vi "RetriggerableHost_20230407.vi"() -> ()   [LabVIEW 2021]
doc: "Use this VI as a template to design an application that acquires data using advanced triggering logic from the NI PXIe-5170R/5171R."
uses:
  <instrlib>/_niInstr/Multirecord Acquisition/Interface/v1/Host/Public/Requested Record Info.ctl
  Controls/Queue_Data_Type.ctl
  <instrlib>/HSAI-RIO/Types/v1/Host/Typedefs/Temp Source.ctl
  <vilib>/FPGAPlugInAG/PXIe-5172 (8CH - 325T)/niLvFpga_Open_PXIe-5172 (8CH - 325T).vi
  <vilib>/rvi/interface/common/dynamic/niFpgaDynamicAddResources.vi
  <vilib>/FPGAPlugInAG/Dynamic/niLvFpga_Close_Dynamic.vi
  <vilib>/rvi/interface/nirviOpenFPGA/nirviOpenFPGA.xnode
  FPGA Bitfiles/Multirecord Acquisition_20220927.lvbitx
  <vilib>/rvi/interface/nirviCloseFPGA/nirviCloseFPGA.xnode
  Device Session/Device Session.lvclass
  <instrlib>/HSAI-RIO/Types/v1/Host/niHSAI Types v1 Host.lvlib
  <vilib>/Utility/TDMS File Viewer/NI_TDMS File Viewer.lvlib
  <instrlib>/_niInstr/Multirecord Acquisition/Interface/v1/Host/niInstr Multirecord Acquisition v1 Host.lvclass
panel:
  out "requested records info":T1[](array[typedef])
  in  "starting record":u64
  out "error out 2":errorcluster
  out "appended path":path
  out "Trigger":bool
  in  "trigger level lo (V)":dbl=-0.25
  in  "trigger level hi (V)":dbl=0.25
  out "actual sample rate":dbl=200000000.0 format="%#_6p"
  in  "onboard sample clock rate":dbl(ring)=200000000.0 items=["250 MHz"=250000000.0, "200 MHz"=200000000.0, "150 MHz"=150000000.0]
  in  "impedance":enum8{"Default", "1 mega ohm", "50 ohm"}(ring)=enum."50 ohm"
  in  "vertical offset (V)":dbl format="%.2p"
  out "Graph":T2(graph)
  out "fpga temperature (°C)":dbl(slide)=84.16040039062506 scale=0.0..96.0 scale format="%#_6p"
  out "power consumption (W)":dbl(slide)=28.75 scale=0.0..38.25 scale format="%#_6p"
  in  "decimation factor":u16=1
  in  "coupling":enum8{"Default", "DC", "AC"}(ring)
  in  "bandwidth":T3(ring)
  in  "pretrigger samples":u64=500
  in  "number of samples":u64=1000
  in  "RIO Device":tag="PXI1Slot2"
  in  "channel(s)":string="0,1"
  in  "vertical range (Vpp)":dbl=1.0 format="%.2p"
  out "error out":errorcluster
  in  "stop":bool
  # "RIO Device"
  # "Vertical Settings"
  # "Trigger Settings"
  # "System Monitor"
  # "Acquisition Settings"
  # "Clocking"
  # "DSP"
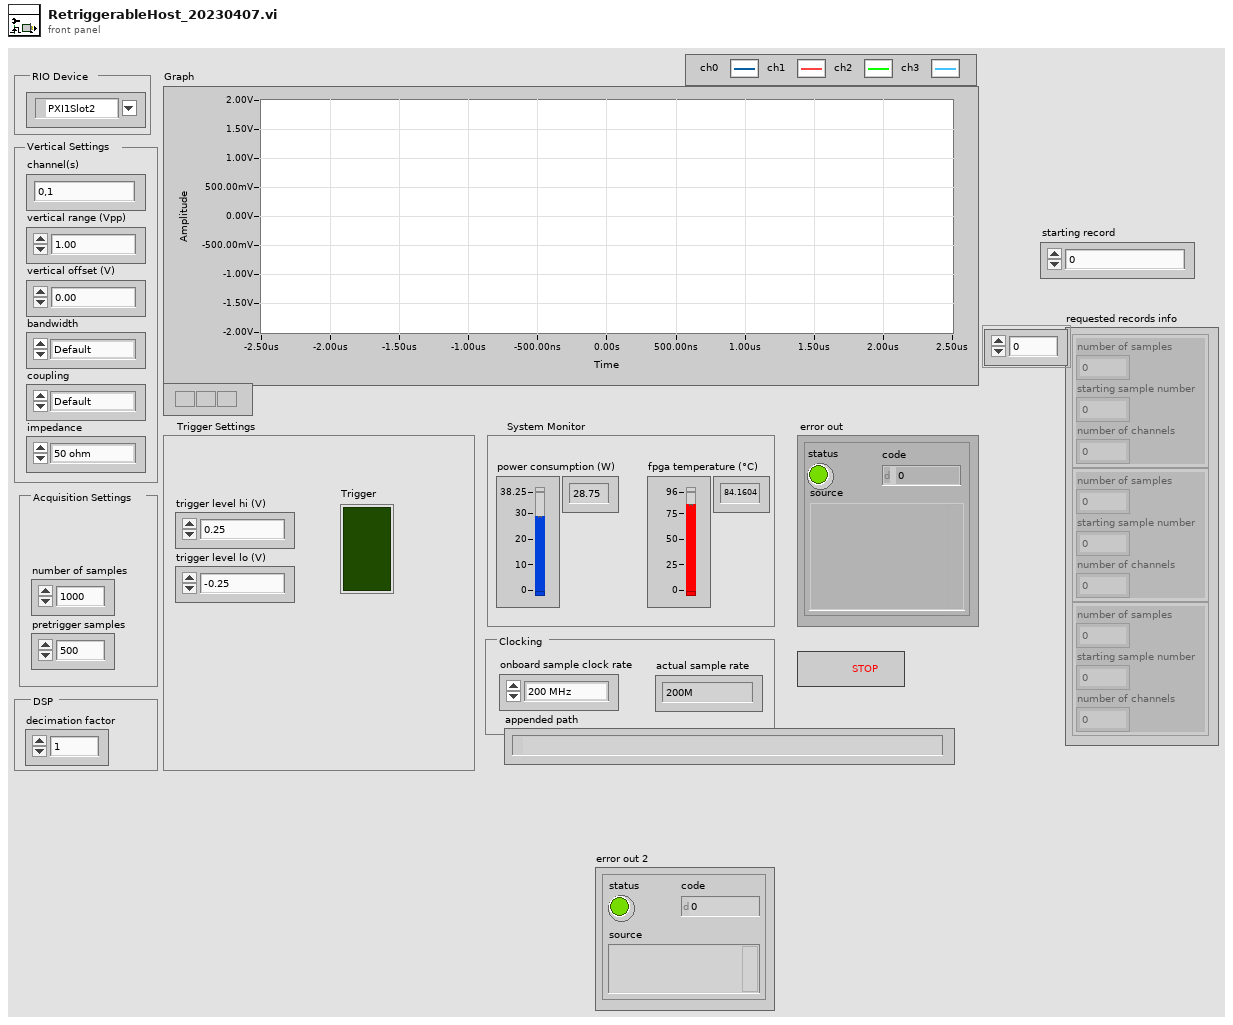
[diagram p1: front panel]
types:
  T1 = typedef "niInstr Multirecord Acquisition v1 Host.lvclass/Requested Record Info.ctl" = cluster{"number of samples":u64, "starting sample number":u64, "number of channels":u64, "timestamps":u64[]}
  T2 = cluster{"relativeX":dbl, "sample rate":dbl, "data in":dbl[]}[]
  T3 = enum8{"Default", "Full Bandwidth", "Anti-alias Filter", "80 MHz FIR Filter", "40 MHz FIR Filter", "20 MHz FIR Filter"}
  T4 = typedef "Queue_Data_Type.ctl" = cluster{"date/time string":string, "data":dbl[][]}
  T5 = enum16{"open", "open or create", "create or replace", "create", "open (read-only)"}
  T6 = enum16{"Immediate", "A", "B", "OR", "AND", "A THEN B", "B THEN A", "High Resolution"}
  T7 = typedef "niHSAI Types v1 Host.lvlib/Temp Source.ctl" = enum8{"Device Temperature", "Thermal Shutdown Margin", "FPGA Temperature", "FPGA Temperature Limit"}
  T8 = cluster{"date/time string":string, "data":dbl[][]}
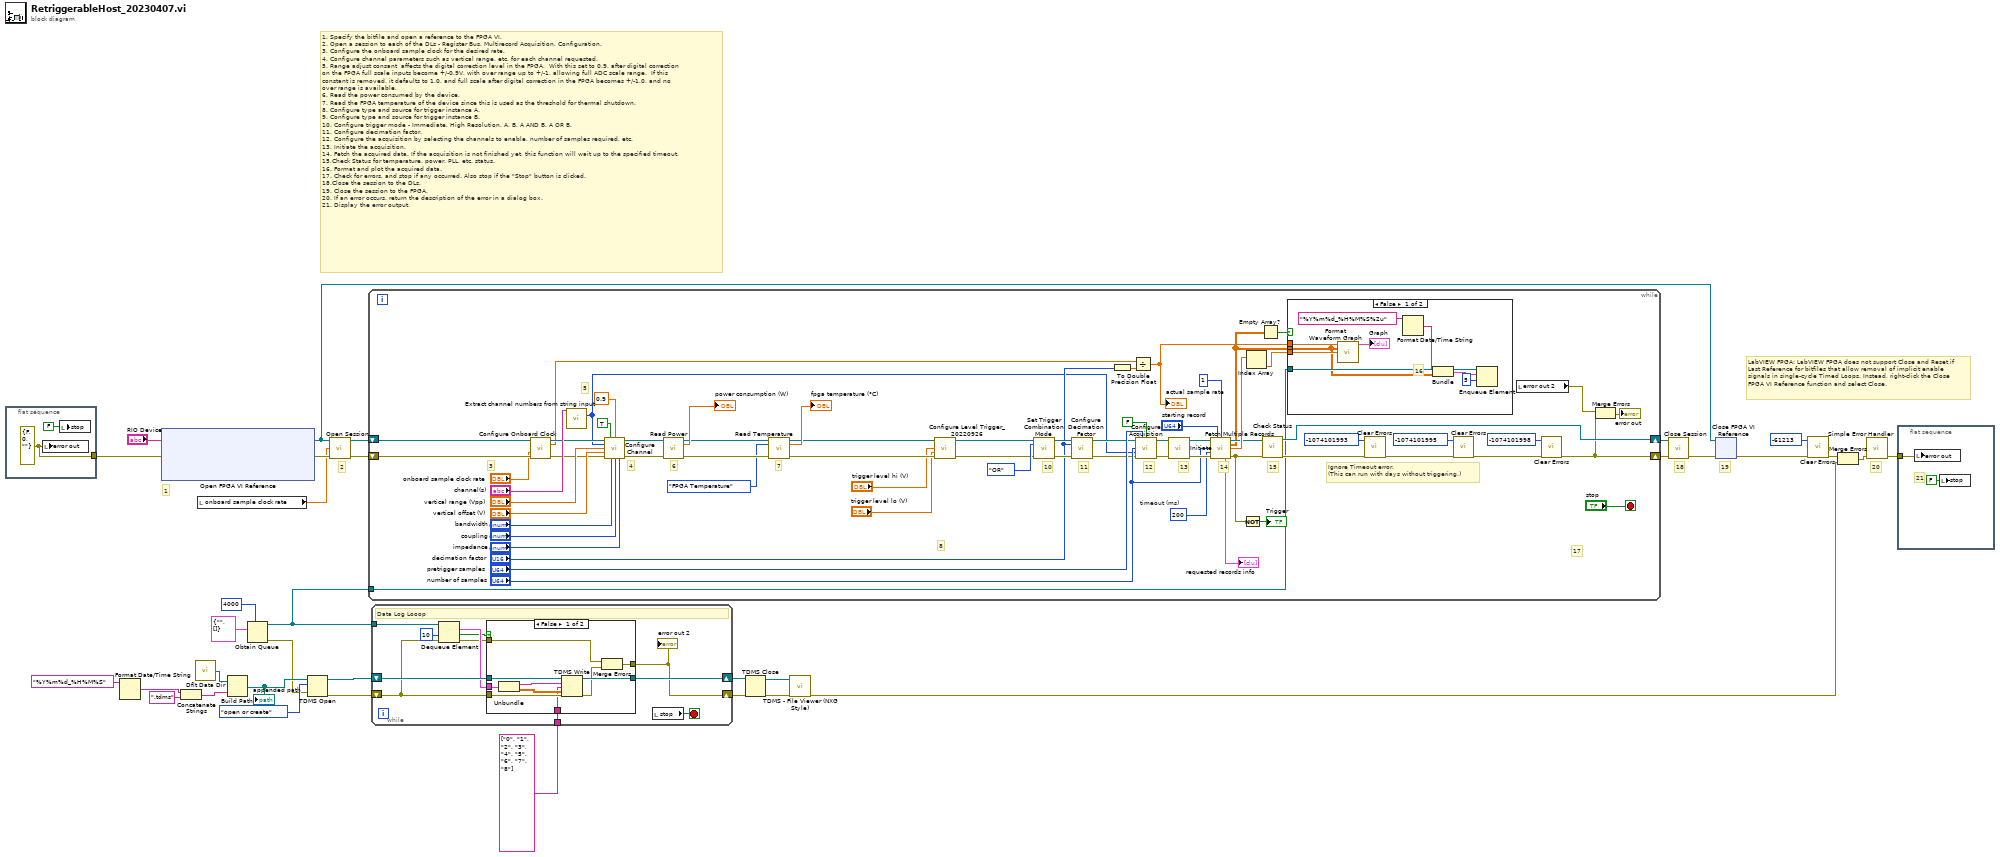
[diagram p0: block diagram]
diagram:
  # "LabVIEW FPGA: LabVIEW FPGA does not support Close and Reset if Last Reference for bitfiles that allow removal of implicit enable signals in single-cycle Timed Loops. Instead, right-click the Close FPGA VI Reference function and select Close."
  # "20"
  # "19"
  # "18"
  # "1. Specify the bitfile and open a reference to the FPGA VI.\n2. Open a session to each of the DLs - Register Bus, Multirecord Acquisition, Configuration.\n3. Configure the onboard sample clock for the desired rate.\n4. Configure channel parameters such as vertical range, etc. for each channel requested.\n5. Range adjust consant  affects the digital correction level in the FPGA.  With this set to 0.9, after digital correction\non the FPGA full scale inputs become +/-0.9V, with over range up to +/-1, allowing full ADC scale range.  If this \nconstant is removed, it defaults to 1.0, and full scale after digital correction in the FPGA becomes +/-1.0, and no\nover range is available.  \n6. Read the power consumed by the device.\n7. Read the FPGA temperature of the device since this is used as the threshold for thermal shutdown.\n8. Configure type and source for trigger instance A.\n9. Configure type and source for trigger instance B.\n10. Configure trigger mode - Immediate, High Resolution, A, B, A AND B, A OR B.\n11. Configure decimation factor.\n12. Configure the acquisition by selecting the channels to enable, number of samples required, etc.\n13. Initiate the acquisition.\n14. Fetch the acquired data. If the acquisition is not finished yet, this function will wait up to the specified timeout.\n15.Check Status for temperature, power, PLL, etc. status. \n16. Format and plot the acquired data.\n17. Check for errors, and stop if any occurred. Also stop if the \"Stop\" button is clicked.\n18.Close the session to the DLs.\n19. Close the session to the FPGA.\n20. If an error occurs, return the description of the error in a dialog box.\n21. Display the error output."
  # "2"
  # "1"
  n1 = flat-sequence {
    tunnel: [w36] -> w24
    frame #0 {
      w36 = errorcluster {"status"=FALSE, "code"=0, "source"=""} ("error out")
      n2 = local write "error out"(w36) -> ()
      n3 = local write "stop"(FALSE ("stop")) -> ()
    }
  }
  n4 = Format Date/Time String(time format string (%c)="%Y%m%d_%H%M%S") -> (date/time string=w22:string)  [unwired: 2 in]
  n5 = xnode "Open FPGA VI Reference"("error in"=w24, "resource name"="RIO Device") -> ("FPGA VI Reference Out"=w27:refnum<k20>, "error out"=w29:errorcluster)
  n6 = Concatenate Strings(w22, ".tdms" ("string")) -> (w21:string)
  n7 = call <vilib>:"Dflt Data Dir.vi"() -> ("App:Default Data Directory"=w23:path)
  n8 = local read "onboard sample clock rate"() -> (w26:dbl)
  n9 = Build Path(base path=w23, name or relative path=w21) -> (appended path=w18:path)
  "appended path" <- w18
  n10 = Obtain Queue(max queue size (-1, unlimited)=4000, element data type=T4 {"date/time string"="", "data"=[]} ("cluster")) -> (queue out=w8:refnum<queue>, error out=w16:errorcluster)  [unwired: 3 in, 1 out]
  n11 = TDMS Open(8:w16, 10:T5."open or create" ("operation (0:open)"), 11:w18) -> (0:w14:errorcluster, 3:w11:refnum<k34>)  [unwired: 4 in]
  n12 = call "Open Session.vi"("fpga reference in"=w27, "adc clock rate (Hz)"=w26, "error in"=w29) -> ("device session out"=w32:refnum<class "Device Session.lvclass">, "error out"=w31:errorcluster)  [unwired: 11 in]
  n13 = while {
    shift-right: [w50] -> w34
    shift-left: w31 -> [w90]
    shift-right: [w55] -> w33
    shift-left: w32 -> [w91]
    tunnel: w8 -> [w45]
    stop <- "stop" stop-if-true
    w38 = 200  # timeout (ms)
    # "Ignore Timeout error.\n(This can run with days without triggering.)"
    # "4"
    # "5"
    # "7"
    # "6"
    # "15"
    # "11"
    # "3"
    # "17"
    # "10"
    # "8"
    # "14"
    # "13"
    # "12"
    n14 = call "Configure Onboard Clock.vi"("device session in"=w91, "adc clock rate (Hz)"="onboard sample clock rate", "error in"=w90) -> ("device session out"=w89:refnum<class "Device Session.lvclass">, "actual adc clock rate (Hz)"=w81:dbl, "error out"=w88:errorcluster)  [unwired: 9 in, 1 out]
    n15 = call "Extract channel numbers from string input.vi"("channel input"="channel(s)") -> ("array of chans"=w61:u32[])  [unwired: 13 in, 1 out]
    n16 = call "Configure Channel.vi"("device session in"=w89, "enable channel (T)"=TRUE ("enable channel"), "range adjust"=0.9, "channels"=w61, "vertical range (Vpp)"="vertical range (Vpp)", "vertical offset (V)"="vertical offset (V)", "error in"=w88, "bandwidth"="bandwidth", "coupling"="coupling", "impedance"="impedance") -> ("device session out"=w73:refnum<class "Device Session.lvclass">, "error out"=w72:errorcluster)  [unwired: 4 in]
    n17 = call "Read Power.vi"("device session in"=w73, "error in"=w72) -> ("device session out"=w74:refnum<class "Device Session.lvclass">, "power (W)"=→"power consumption (W)":dbl, "error out"=w75:errorcluster)  [unwired: 11 in]
    n18 = call "Read Temperature.vi"("device session in"=w74, "source"=Temp_Source."FPGA Temperature", "error in"=w75) -> ("device session out"=w71:refnum<class "Device Session.lvclass">, "temperature (°C)"=→"fpga temperature (°C)":dbl, "error out"=w70:errorcluster)  [unwired: 10 in]
    n19 = call "Configure Level Trigger_20220926.vi"("device session in"=w71, "trigger level hi (V)"="trigger level hi (V)", "trigger level lo (V)"="trigger level lo (V)", "error in"=w70) -> ("device session out"=w60:refnum<class "Device Session.lvclass">, "error out"=w59:errorcluster)  [unwired: 10 in]
    n20 = call "Set Trigger Combination Mode.vi"("device session in"=w60, "mode"=T6."OR", "error in"=w59) -> ("device session out"=w86:refnum<class "Device Session.lvclass">, "error out"=w85:errorcluster)  [unwired: 11 in]
    n21 = call "Configure Decimation Factor.vi"("device session in"=w86, "decimation factor"="decimation factor", "error in"=w85) -> ("device session out"=w83:refnum<class "Device Session.lvclass">, "error out"=w84:errorcluster)  [unwired: 11 in]
    n22 = To Double Precision Float(number="decimation factor") -> (double precision float=w87:dbl)
    n23 = Divide(x=w81, y=w87) -> (x/y=w63:dbl)
    "actual sample rate" <- w63
    n24 = call "Configure Acquisition.vi"("device session in"=w83, "pretrigger samples"="pretrigger samples", "number of records is finite (T)"=FALSE, "number of samples"="number of samples", "channels to store"=w61, "error in"=w84) -> ("device session out"=w98:refnum<class "Device Session.lvclass">, "error out"=w101:errorcluster)  [unwired: 7 in, 1 out]
    n25 = call "Initiate.vi"("device session in"=w98, "error in"=w101) -> ("device session out"=w99:refnum<class "Device Session.lvclass">, "error out"=w100:errorcluster)  [unwired: 12 in]
    n26 = call "Fetch Multiple Records.vi"("device session in"=w99, "starting record"="starting record", "number of records"=u64 1, "number of samples"="number of samples", "timeout (ms)"=w38, "error in"=w100) -> ("device session out"=w78:refnum<class "Device Session.lvclass">, "data"=w47:dbl[][], "relativeX (samples)"=w92:dbl[], "requested records info"=→"requested records info":T1[], "error out"=w48:errorcluster)  [unwired: 5 in]
    n27 = Not(x=w48) -> (.not. x?=→"Trigger":bool)
    n28 = Index Array(array=w92) -> (element=w39:dbl)  [unwired: 1 in]
    n29 = Empty Array?(array=w47) -> (empty?=w46:bool)
    n30 = call "Check Status.vi"("device session in"=w78, "error in"=w48) -> ("device session out"=w55:refnum<class "Device Session.lvclass">, "error out"=w79:errorcluster)  [unwired: 12 in]
    n31 = case shown="False" w46 {
      tunnel: w47 -> [w107 _]
      tunnel: w39 -> [w111 _]
      tunnel: w63 -> [w109 _]
      tunnel: w45 -> [w108 _]
      frame False {
        # "16"
        n32 = call "Format Waveform Graph.vi"("sample rate (Hz)"=w109, "data in"=w107, "relativeX (samples)"=w111) -> ("waveform out"=→"Graph":T2)  [unwired: 12 in]
        n33 = Format Date/Time String(time format string (%c)="%Y%m%d_%H%M%S%2u") -> (date/time string=w103:string)  [unwired: 2 in]
        n34 = Bundle("date/time string"=w103, "data"=w107) -> (w104:T8)  [unwired: 1 in]
        n35 = Enqueue Element(queue=w108, element=w104, timeout in ms (-1)=5) -> ()  [unwired: 1 in, 3 out]
      }
      frame True {
        # "No data"
      }
    }
    n36 = call <vilib>:"Clear Errors.vi"("error in (no error)"=w79, "specific error code to clear (0: all)"=-1074101993) -> ("error out"=w53:errorcluster)  [unwired: 4 in, 1 out]
    n37 = call <vilib>:"Clear Errors.vi"("error in (no error)"=w53, "specific error code to clear (0: all)"=-1074101995) -> ("error out"=w51:errorcluster)  [unwired: 4 in, 1 out]
    n38 = local read "error out 2"() -> (w43:errorcluster)
    n39 = call <vilib>:"Clear Errors.vi"("error in (no error)"=w51, "specific error code to clear (0: all)"=-1074101998) -> ("error out"=w50:errorcluster)  [unwired: 4 in, 1 out]
    n40 = Merge Errors(w43, w50) -> (→"error out":errorcluster)
  }
  n41 = while {
    shift-right: [w114] -> w13
    shift-left: w14 -> [w119]
    shift-right: [w121] -> w10
    shift-left: w11 -> [w122]
    tunnel: w8 -> [w120]
    tunnel: string[] ["0", "1", "2", "3", "4", "5", "6", "7", "8"] ("channel name(s) in (Untitled)") -> [w112]
    stop <- w116 stop-if-true
    # "Data Log Looop"
    n42 = Dequeue Element(queue=w120, timeout in ms (-1)=10, error in (no error)=w119) -> (element=w118:T4, timed out?=w113:bool, error out=w117:errorcluster)  [unwired: 1 out]
    n43 = case shown="False" w113 {
      tunnel: w122 -> [w132 w134]
      tunnel: [w131 w134] -> w121
      tunnel: w119 -> [w130 _]
      tunnel: w118 -> [w129 _]
      tunnel: w117 -> [w128 w133]
      tunnel: [w126 w133] -> w114
      tunnel: w112 -> [w123 _]
      frame False {
        n44 = Unbundle(w129) -> ("date/time string"=w125:string, "data"=w124:dbl[][])
        n45 = TDMS Write(0:w132, 5:w125, 7:w123, 9:w124, 11:w130) -> (4:w131:refnum<k34>, 15:w127:errorcluster)  [unwired: 1 in, 2 out]
        n46 = Merge Errors(w128, w127) -> (w126:errorcluster)
      }
      frame True {
        # "Timed out. No data."
      }
    }
    "error out 2" <- w114
    n47 = local read "stop"() -> (w116:bool)
  }
  n48 = TDMS Close(8:w13, 11:w10) -> (0:w12:errorcluster, 3:w9:path)
  n49 = call <vilib>:"TDMS - File Viewer (NXG Style).vi"("error in"=w12, "file in"=w9) -> ("error out"=w6:errorcluster)  [unwired: 8 in, 1 out]
  n50 = call "Close Session.vi"("device session in"=w33, "error in"=w34) -> ("error out"=w28:errorcluster)  [unwired: 13 in]
  n51 = xnode "Close FPGA VI Reference"("FPGA VI Reference In"=w27, "error in"=w28) -> ("error out"=w2:errorcluster)
  n52 = call <vilib>:"Clear Errors.vi"("error in (no error)"=w2, "specific error code to clear (0: all)"=-61213) -> ("error out"=w1:errorcluster)  [unwired: 4 in, 1 out]
  n53 = Merge Errors(w1, w6) -> (w7:errorcluster)
  n54 = call <vilib>:"Simple Error Handler.vi"("error in (no error)"=w7) -> ("error out"=w25:errorcluster)  [unwired: 4 in, 4 out]
  n55 = flat-sequence {
    tunnel: w25 -> [w136]
    frame #0 {
      # "21"
      n56 = local write "error out"(w136) -> ()
      n57 = local write "stop"(FALSE ("stop")) -> ()
    }
  }
